vi "labHolo.vi"() -> ()   [LabVIEW 2023] (continued)
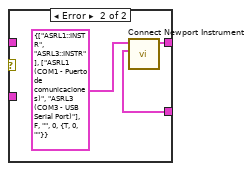
[diagram p2: hidden frame]
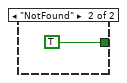
[diagram p4: hidden frame]
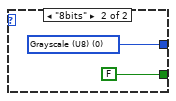
[diagram p5: hidden frame]
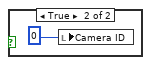
[diagram p6: hidden frame]
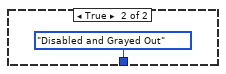
[diagram p7: hidden frame]
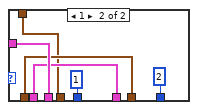
[diagram p8: hidden frame]
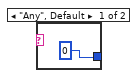
[diagram p13: hidden frame]
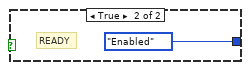
[diagram p14: hidden frame]
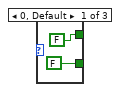
[diagram p15: hidden frame]
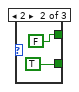
[diagram p16: hidden frame]
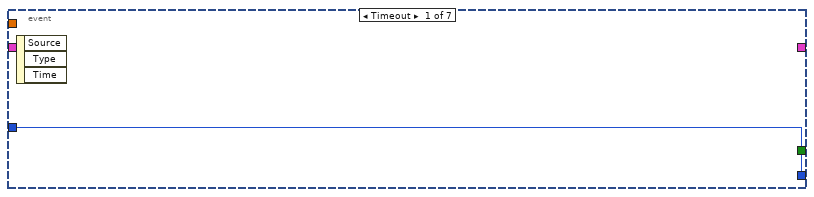
[diagram p17: hidden frame]
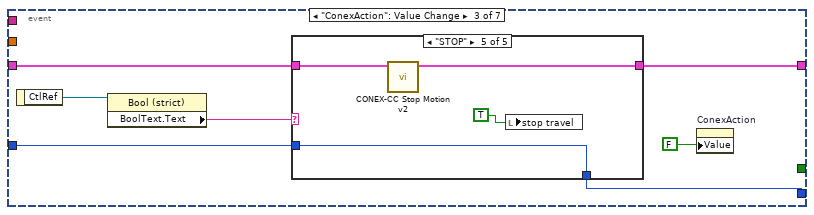
[diagram p18: hidden frame]
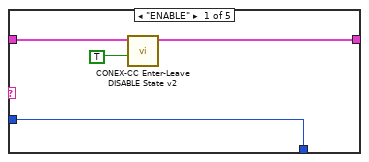
[diagram p19: hidden frame]
                n313 = Unbundle By Name(w777) -> ("1_Ygros"=w782:dbl, "1_Yfine"=w783:dbl)
                n314 = Multiply(x=w781, y=w782) -> (x*y=w780:dbl)
                n315 = Multiply(x=w783, y=w781) -> (x*y=w778:dbl)
                n316 = property on="Ygros" class="Slide (strict)"("Val(Sgnl)"=w780) -> (error out=w779:errorcluster)  [unwired: 2 in, 1 out]
                n317 = Bundle By Name(cluster=w777, "1_Ygros"=w780, "1_Yfine"=w778, "1_Yreverse"=w775) -> (w776:T4)
                n318 = property on="Yfine" class="Slide (strict)"(error in=w779, "Val(Sgnl)"=w778) -> ()  [unwired: 1 in, 2 out]
              }
            }
            n319 = case shown="1" w724 {
              tunnel: w729 -> [w733 w735]
              tunnel: w731 -> [w732 w734]
              frame 0, Default {
                n320 = local write "1_posCluster"(w733) -> ()
                n321 = local write "1_mainPos"(w732) -> ()
              }
              frame 1 {
                n322 = local write "2_posCluster"(w735) -> ()
                n323 = local write "2_mainPos"(w734) -> ()
              }
            }
          }
          event "setXi", "setXf", "setYi", "setYf": Value Change {
            w788 = FALSE ("setYf")
            n324 = event-data() -> ("CtlRef"=w787:refnum<vi>)  [unwired: 1 in, 2 out]
            n325 = case shown="0, Default" w786 {
              tunnel: [w804 w805] -> w790
              frame 0, Default {
                n326 = local read "1_mainPos"() -> (w804:T3)
              }
              frame 1 {
                n327 = local read "2_mainPos"() -> (w805:T3)
              }
            }
            n328 = property class="Bool (strict)"(reference=w787) -> ("Label.Text"=w789:string)  [unwired: 1 in, 2 out]
            n329 = local read "Ypos"() -> (w792:i32)
            n330 = local read "Xpos"() -> (w791:i32)
            n331 = case shown="\"setYf\"" w789 {
              tunnel: w790 -> [w808 w811 w813 w816 w819]
              tunnel: [w808 w810 w812 w815 w818] -> w793
              tunnel: w791 -> [_ w809 w814 _ _]
              tunnel: w792 -> [_ _ _ w817 w820]
              frame "Any", Default {
              }
              frame "setXi" {
                n332 = Bundle By Name(cluster=w811, "1_Xi"=w809) -> (w810:T3)
              }
              frame "setXf" {
                n333 = Bundle By Name(cluster=w813, "1_Xf"=w814) -> (w812:T3)
              }
              frame "setYi" {
                n334 = Bundle By Name(cluster=w816, "1_Yi"=w817) -> (w815:T3)
              }
              frame "setYf" {
                n335 = Bundle By Name(cluster=w819, "1_Yf"=w820) -> (w818:T3)
              }
            }
            n336 = Unbundle By Name(w793) -> ("1_Xi"=w795:dbl, "1_Xf"=w796:dbl, "1_Yi"=w797:dbl, "1_Yf"=w798:dbl)
            n337 = local write "setYf"(w788) -> ()
            n338 = local write "setYi"(w788) -> ()
            n339 = local write "setXf"(w788) -> ()
            n340 = local write "setXi"(w788) -> ()
            n341 = call "pos2centerRadi.vi"("pos fin"=w796, "pos init"=w795) -> ("semi diff (r)"=w802:dbl, "semi sum (C)"=w803:dbl)  [unwired: 8 in]
            n342 = call "pos2centerRadi.vi"("pos fin"=w798, "pos init"=w797) -> ("semi diff (r)"=w800:dbl, "semi sum (C)"=w801:dbl)  [unwired: 8 in]
            n343 = Divide(x=w802, y=w800) -> (x/y=w799:dbl)
            n344 = Bundle By Name(cluster=w793, "1_Xcenter"=w803, "1_Diam. X"=w802, "1_Ycenter"=w801, "1_Diam. Y"=w800, "1_Form fa."=w799) -> (w794:T3)
            n345 = local write "Form fa."(w799) -> ()
            n346 = local write "Diam. Y"(w800) -> ()
            n347 = local write "Ycenter"(w801) -> ()
            n348 = local write "Diam. X"(w802) -> ()
            n349 = local write "Xcenter"(w803) -> ()
            n350 = case shown="1" w786 {
              tunnel: w794 -> [w806 w807]
              frame 0, Default {
                n351 = local write "1_mainPos"(w806) -> ()
              }
              frame 1 {
                n352 = local write "2_mainPos"(w807) -> ()
              }
            }
          }
          event "SLM_number": Value Change {
            n353 = event-data() -> ("NewVal"=w825:u16)  [unwired: 1 in]
            n354 = case shown="1" w825 {
              tunnel: [w860 w863] -> w855
              tunnel: [w859 w862] -> w839
              tunnel: [w858 w861] -> w849
              frame 0, Default {
                n355 = local read "1_posCluster"() -> (w859:T4)
                n356 = local read "SLM1 cluster"() -> (w860:T2)
                n357 = local read "1_mainPos"() -> (w858:T3)
              }
              frame 1 {
                n358 = local read "SLM2 cluster"() -> (w863:T2)
                n359 = local read "2_posCluster"() -> (w862:T4)
                n360 = local read "2_mainPos"() -> (w861:T3)
              }
            }
            n361 = Unbundle By Name(w855) -> ("1_Radio"=w823:T7, "1_Trans"=w829:dbl, "1_Phase"=w830:dbl, "1_HoloCode"=w831:string, "1_Semi"=w832:bool, "1_Active"=w857:u16, "1_ModType"=w833:string, "1_Flip"=w834:string, "1_HoloNum"=w835:dbl, "1_key1"=w836:string, "1_value1"=w837:i64, "1_key2"=w838:string)
            n362 = Unbundle By Name(w849) -> ("1_Xcenter"=w850:dbl, "1_Ycenter"=w851:dbl, "1_Diam. X"=w852:dbl, "1_Diam. Y"=w853:dbl, "1_Form fa."=w854:dbl)
            n363 = Unbundle By Name(w839) -> ("1_Xoffset"=w840:dbl, "1_Yoffset"=w841:dbl, "1_Xgros"=w842:dbl, "1_Ygros"=w843:dbl, "1_Xfine"=w844:dbl, "1_Yfine"=w845:dbl, "1_Xreverse"=w846:u16, "1_Yreverse"=w847:u16, "1_XYswap"=w848:u16)
            n364 = local write "Radio"(w823) -> ()
            n365 = local write "Trans"(w829) -> ()
            n366 = local write "Phase"(w830) -> ()
            n367 = local write "HoloCode"(w831) -> ()
            n368 = local write "Semi"(w832) -> ()
            n369 = local write "Active"(w857) -> ()
            n370 = local write "ModType"(w833) -> ()
            n371 = local write "Flip"(w834) -> ()
            n372 = local write "HoloNum"(w835) -> ()
            n373 = local write "Xreverse"(w846) -> ()
            n374 = local write "Yreverse"(w847) -> ()
            n375 = local write "XYswap"(w848) -> ()
            n376 = local write "Xcenter"(w850) -> ()
            n377 = local write "Ycenter"(w851) -> ()
            n378 = local write "Diam. X"(w852) -> ()
            n379 = local write "Diam. Y"(w853) -> ()
            n380 = local write "Form fa."(w854) -> ()
            n381 = local write "Xoffset"(w840) -> ()
            n382 = local write "Ygros"(w843) -> ()
            n383 = local write "Xfine"(w844) -> ()
            n384 = local write "value1"(w837) -> ()
            n385 = local write "Yoffset"(w841) -> ()
            n386 = local write "Xgros"(w842) -> ()
            n387 = local write "Yfine"(w845) -> ()
            n388 = local write "key1"(w836) -> ()
            n389 = local write "key2"(w838) -> ()
            n390 = Increment(x=w825) -> (x+1=w856:u16)
            n391 = call "holoPathEditor.vi"("Display"=w856, "prev. Path"=w826, "input cluster"=w855) -> ("appended path"=w827:path)  [unwired: 5 in, 3 out]
            n392 = Unbundle(w822) -> ("New Image"=w821:T6)  [unwired: 2 out]
            n393 = call "IMAQ ReadFile"("File Path"=w827, "Image"=w821) -> ("Image Out"=w828:T6)  [unwired: 5 in, 4 out]
            n394 = property on="Active" class="Ring (strict)"("Val(Sgnl)"=w857) -> ()  [unwired: 2 in, 2 out]
          }
          event "Parada Total": Value Change {
            n395 = event-data() -> ("NewVal"=w868:bool)  [unwired: 1 in, 5 out]
            n396 = Close Python Session(session in=w864) -> ()  [unwired: 1 in, 1 out]
          }
        }
        n397 = local write "CGH path"(w559) -> ()
        n398 = local write "monitor2"(w560) -> ()
        n399 = local write "monitor1"(w560) -> ()
        "error get holo" <- w561
      }
      n400 = while {
        shift-right: [w442] -> _
        shift-left: w318 -> [w443]
        tunnel: w311 -> [w438]
        stop <- w432 stop-if-true
        # "Buttons loop"
        n401 = local read "Last mov."() -> (w439:u16)
        n402 = local read "lambda"() -> (w440:dbl)
        n403 = local read "Units"() -> (w441:string)
        n404 = event shown="[1] \"Parada Total\": Value Change" {
          selector: _ -> [_ _ _ _ _ _ _]
          dyn-events: _ -> [_ _ _ _ _ _ _]
          timeout: _ -> [_ _ _ _ _ _ _]
          tunnel: [_ w453 _ _ _ _ _] -> w432
          tunnel: w443 -> [_ w454 w472 w506 w526 w533 w544]
          tunnel: [_ w452 w471 w505 w525 w533 w544] -> w442
          tunnel: w441 -> [_ _ _ w499 w524 _ _]
          tunnel: w440 -> [_ _ _ w498 w523 _ w537]
          tunnel: [w450 w451 w467 w496 w515 w532 w536] -> w437
          tunnel: w439 -> [w450 w451 w466 _ _ w532 w536]
          tunnel: w438 -> [_ _ _ w497 _ _ _]
          event Timeout {
            n405 = event-data() -> ()  [unwired: 1 in, 3 out]
          }
          event "Parada Total": Value Change {
            n406 = event-data() -> ()  [unwired: 1 in, 1 out]
            n407 = flat-sequence {
              tunnel: [w459] -> w457
              tunnel: w454 -> [w458]
              tunnel: w457 -> [w461]
              tunnel: [w461] -> w456
              tunnel: w456 -> [w463]
              tunnel: [w463] -> w455
              tunnel: [w465] -> w452
              tunnel: w455 -> [w465]
              tunnel: [TRUE] -> w453
              frame #0 {
                n408 = call "CONEX-CC Stop Motion v2.vi"("Connection Cluster in"=w458) -> ("Connection Cluster out"=w459:T16)  [unwired: 10 in]
              }
              frame #1 {
                n409 = local write "Travel"(FALSE) -> ()
              }
              frame #2 {
                n410 = Wait (ms)(milliseconds to wait=u32 200 ("attente (ms)")) -> ()  [unwired: 1 out]
              }
              frame #3 {
              }
            }
          }
          event "ConexAction": Value Change {
            n411 = event-data() -> ("CtlRef"=w469:refnum<vi>)  [unwired: 1 in]
            n412 = property on="Property Node" class="Bool (strict)"(reference=w469) -> ("BoolText.Text"=w468:string)  [unwired: 1 in, 2 out]
            n413 = case shown="\"STOP\"" w468 {
              tunnel: w472 -> [w475 w478 w481 w489 w492]
              tunnel: [w474 w478 w480 w488 w493] -> w471
              tunnel: [w473 w477 w479 w486 w491] -> w467
              tunnel: w466 -> [w473 w477 _ w486 w491]
              frame "ENABLE" {
                n414 = call "CONEX-CC Enter-Leave DISABLE State v2.vi"("Ready? (false=DISABLE true=READY)"=TRUE ("Flag (false=DISABLE true=READY)"), "Connection Cluster in"=w475) -> ("Connection Cluster out"=w474:T16)  [unwired: 7 in]
              }
              frame Default {
              }
              frame "HOME" {
                n415 = flat-sequence {
                  tunnel: w481 -> [w485]
                  tunnel: [w484] -> w480
                  tunnel: [w483] -> w479
                  frame #0 {
                    n416 = One Button Dialog(message="The Stage will go to the 0 position. Check that the travel is clean!") -> ()  [unwired: 1 in, 1 out]
                  }
                  frame #1 {
                    w483 = u16 0 items=["opening", "homing", "toLeft", "toRight", "closing"] ("Last movement")
                    n417 = call "CONEX-CC Home search v2.vi"("Connection Cluster in"=w485) -> ("Connection Cluster out"=w484:T16)  [unwired: 5 in, 3 out]
                  }
                }
              }
              frame "DISABLE" {
                n418 = call "CONEX-CC Enter-Leave DISABLE State v2.vi"("Ready? (false=DISABLE true=READY)"=FALSE ("Flag (false=DISABLE true=READY)"), "Connection Cluster in"=w489) -> ("Connection Cluster out"=w488:T16)  [unwired: 7 in]
              }
              frame "STOP" {
                n419 = call "CONEX-CC Stop Motion v2.vi"("Connection Cluster in"=w492) -> ("Connection Cluster out"=w493:T16)  [unwired: 10 in]
                n420 = local write "stop travel"(TRUE ("stop travel")) -> ()
              }
            }
            n421 = property on="ConexAction" class="Bool (strict)"("Value"=FALSE) -> ()  [unwired: 2 in, 2 out]
          }
          event "step forward", "step backward": Value Change {
            n422 = event-data() -> ("CtlRef"=w508:refnum<vi>)  [unwired: 1 in]
            n423 = property on="Property Node" class="Bool (strict)"(reference=w508) -> (reference out=w501:refnum<vi>, error out=w503:errorcluster, "Label.Text"=w504:string)  [unwired: 1 in]
            n424 = local read "Step:"() -> (w500:dbl)
            n425 = call "step_movement.vi"("lambda (nm)"=w498, "Units"=w499, "error in (no error)"=w503, "step (units)"=w500, "Step type (fordward)"=w504, "Connection Cluster in"=w506) -> ("error out"=w502:errorcluster, "Last mov."=w496:u16, "Connection Cluster out"=w505:T16)  [unwired: 3 in]
            n426 = property on="Property Node" class="Bool (strict)"(reference=w501, error in=w502, "Value"=FALSE) -> (error out=w495:errorcluster)  [unwired: 1 out]
            n427 = local read "Travel"() -> (w494:bool)
            n428 = case shown="True" w494 {
              tunnel: w497 -> [_ w511]
              tunnel: w495 -> [_ w510]
              frame False {
              }
              frame True {
                n429 = Send Notification(notification="", notifier=w511, error in (no error)=w510) -> ()  [unwired: 2 out]
              }
            }
          }
          event "Go1", "Go2", "Go0": Value Change {
            n430 = event-data() -> ("CtlRef"=w522:refnum<vi>)  [unwired: 1 in]
            n431 = property on="Property Node" class="Bool (strict)"(reference=w522) -> (reference out=w521:refnum<vi>, "Label.Text"=w519:string)  [unwired: 1 in, 1 out]
            n432 = case shown="\"Go0\", Default" w519 {
              tunnel: [w529 w530 0.0 ("(2) Go to:")] -> w513
              frame "Go1" {
                n433 = local read "(1) Go to:"() -> (w529:dbl)
              }
              frame "Go2" {
                n434 = local read "(2) Go to:"() -> (w530:dbl)
              }
              frame "Go0", Default {
              }
            }
            n435 = local read "Zero pos."() -> (w514:dbl)
            n436 = Add(x=w514, y=w513) -> (x+y=w512:dbl)
            n437 = local read "Relative pos."() -> (w517:dbl)
            n438 = call "units2mm.vi"("lambda (nm)"=w523, "target units"=w524, "position in units"=w512) -> ("raw postion (mm)"=w518:dbl)  [unwired: 8 in]
            n439 = property on="Property Node" class="Bool (strict)"(reference=w521, "Value"=FALSE) -> ()  [unwired: 1 in, 2 out]
            n440 = Greater?(x=w518, y=w517) -> (0:w516:bool)
            n441 = case shown="False" w516 {
              tunnel: [w527 w528] -> w515
              frame False {
                w527 = u16 2 items=["opening", "homing", "toLeft", "toRight", "closing"] ("Last movement")
              }
              frame True {
                w528 = u16 3 items=["opening", "homing", "toLeft", "toRight", "closing"] ("Last movement")
              }
            }
            n442 = call "CONEX-CC Absolute Move v2.vi"("Target position"=w518, "Connection Cluster in"=w526) -> ("Connection Cluster out"=w525:T16)  [unwired: 5 in, 2 out]
          }
          event "Tare": Value Change {
            n443 = event-data() -> ()  [unwired: 1 in, 2 out]
            n444 = local read "Raw position"() -> (w535:dbl)
            n445 = local write "Tare"(FALSE ("Tare")) -> ()
            n446 = local write "Zero pos."(w535) -> ()
          }
          event "Units": Value Change {
            n447 = event-data() -> ("OldVal"=w543:string, "NewVal"=w545:string)  [unwired: 1 in]
            n448 = property on="(1) Go to:" class="DigNum (strict)"("Caption.Text"=w545) -> ()  [unwired: 2 in, 2 out]
            n449 = property on="(2) Go to:" class="DigNum (strict)"("Caption.Text"=w545) -> ()  [unwired: 2 in, 2 out]
            n450 = property on="Zero pos." class="DigNum (strict)"("Caption.Text"=w545) -> ()  [unwired: 2 in, 2 out]
            n451 = property on="Raw position" class="DigNum (strict)"("Caption.Text"=w545) -> ()  [unwired: 2 in, 2 out]
            n452 = property on="Relative pos." class="DigNum (strict)"("Caption.Text"=w545) -> ()  [unwired: 2 in, 2 out]
            n453 = property on="Step:" class="DigNum (strict)"("Caption.Text"=w545) -> ()  [unwired: 2 in, 2 out]
            n454 = case shown="\"lam\"" w543 {
              tunnel: [1000000.0 1000.0 1.0 w549] -> w539
              tunnel: w537 -> [_ _ _ w549]
              frame "mm", Default {
              }
              frame "um" {
              }
              frame "nm" {
              }
              frame "lam" {
              }
            }
            n455 = case shown="\"lam\"" w545 {
              tunnel: [1000000.0 1000.0 1.0 w553] -> w538
              tunnel: w537 -> [_ _ _ w553]
              frame "mm", Default {
              }
              frame "um" {
              }
              frame "nm" {
              }
              frame "lam" {
              }
            }
            n456 = local read "Zero pos."() -> (w542:dbl)
            n457 = Divide(x=w539, y=w538) -> (x/y=w540:dbl)
            n458 = Multiply(x=w542, y=w540) -> (x*y=w541:dbl)
            n459 = local write "Zero pos."(w541) -> ()
          }
        }
        n460 = case shown="3" w437 {
          tunnel: [FALSE ("Boolean Text.Font:Bold") FALSE ("Boolean Text.Font:Bold") TRUE ("Boolean Text.Font:Bold")] -> w435
          tunnel: [FALSE ("Boolean Text.Font:Bold") TRUE ("Boolean Text.Font:Bold") FALSE ("Boolean Text.Font:Bold")] -> w436
          frame 0, Default {
          }
          frame 2 {
          }
          frame 3 {
          }
        }
        n461 = Not(x=w432) -> (.not. x?=w431:bool)
        n462 = local write "Last mov."(w437) -> ()
        n463 = And(x=w435, y=w431) -> (x .and. y?=w434:bool)
        n464 = And(x=w436, y=w431) -> (x .and. y?=w433:bool)
        n465 = property on="step backward" class="Bool (strict)"("BoolText.FontUnder"=w433) -> ()  [unwired: 2 in, 2 out]
        n466 = property on="step forward" class="Bool (strict)"("BoolText.FontUnder"=w434) -> ()  [unwired: 2 in, 2 out]
      }
      n467 = while {
        shift-right: [w884] -> _
        shift-left: _ -> [w883]
        tunnel: w330 -> [w881]
        tunnel: w305 -> [w880]
        tunnel: w329 -> [w878]
        tunnel: w328 -> [w877]
        shift-right: [w873] -> _
        shift-left: w327 -> [w875]
        shift-right: [w872] -> _
        shift-left: w326 -> [w874]
        tunnel: w325 -> [w871]
        tunnel: w309 -> [w870]
        tunnel: w310 -> [w869]
        stop <- w885 stop-if-true
        # "Cam control"
        # "pyError"
        # "Reff"
        # "ROI"
        # "CCD"
        # "pySession"
        n468 = local read "Camera ID"() -> (w876:u16)
        n469 = event shown="[0] Timeout" {
          selector: _ -> [_ _ _ _ _ _ _]
          dyn-events: _ -> [_ _ _ _ _ _ _]
          timeout: 10 -> [_ _ _ _ _ _ _]
          tunnel: [_ _ _ _ _ _ w1053] -> w885
          tunnel: [w912 _ _ _ _ _ _] -> w884
          tunnel: w883 -> [w920 _ _ _ _ _ _]
          tunnel: w881 -> [w918 _ _ w963 _ _ _]
          tunnel: w880 -> [w917 _ _ w962 w1005 _ w1052]
          tunnel: [w916 _ _ w961 w1003 _ w1050] -> w879
          tunnel: w878 -> [w901 _ _ _ _ _ _]
          tunnel: w877 -> [w900 _ _ _ _ _ _]
          tunnel: w876 -> [w902 _ _ _ w994 _ _]
          tunnel: w875 -> [w897 _ _ _ _ _ _]
          tunnel: w874 -> [w896 _ _ _ _ _ _]
          tunnel: [w895 _ _ _ _ _ _] -> w873
          tunnel: [w894 _ _ _ _ _ _] -> w872
          tunnel: w871 -> [w892 _ _ w959 w993 _ w1051]
          tunnel: w870 -> [_ _ _ w956 _ _ _]
          tunnel: w869 -> [_ _ _ w954 _ _ _]
          event Timeout {
            n470 = event-data() -> ()  [unwired: 1 in, 3 out]
            n471 = call "capture.vi"("error in (no error)"=w892, "Cam ID"=w902, "Image in"=w918, "session in"=w917) -> ("error out"=w916:errorcluster, "Image out"=w899:T6)  [unwired: 3 in, 1 out]
            n472 = local read "bit depth"() -> (w906:enum16{"16bits", "14bits", "12bits", "8bits"})
            n473 = property on="CCD Image" class="ImageControl"() -> ("ROI"=w886:T8)  [unwired: 2 in, 2 out]
            "ROI" <- w886
            n474 = call "histogram.vi"("Image ROI"=w900, "useROI"="Whole/ROI", "ROI Descriptor"=w886, "bit depth"=w906, "Image"=w899) -> ("Statistics"=w909:T20, "Histograph"=→"Histograph":T9, "bins"=w898:i32)  [unwired: 2 in, 2 out]
            n475 = Unbundle By Name(w909) -> ("mean (ROI)"=w889:dbl, "max (ROI)"=w888:i16, "max_counts"=w908:dbl, "image_size"=→"ROI size":i32, "# Sat. Pixels"=w887:sgl)
            "mean bar" <- w889
            "mean" <- w889
            "max" <- w888
            "# Sat. Pixels" <- w887
            n476 = control-ref of="Histograph"() -> (w907:refnum<vi>)
            n477 = control-ref of="Reff ROI"() -> (w910:refnum<vi>)
            n478 = call "setHistogram.vi"("Auto. In"="Auto. hist", "max counts"=w908, "bins"=w898, "WaveformGraph in"=w907) -> ()  [unwired: 7 in, 1 out]
            n479 = call "drawRoi.vi"("bit depth"=w906, "ROI"=w910, "Reff image"=w901, "Whole image"=w899) -> ("size"=→"size":i32, "mean"=w905:dbl, "Image Out"=w891:T6, "Percentile alert"=w893:bool)  [unwired: 3 in, 1 out]
            "CCD Image" <- w891
            n480 = Tick Count (ms)() -> (millisecond timer value=w912:u32)
            n481 = Subtract(x=w912, y=w920) -> (x-y=w923:u32)
            n482 = case shown="True" "EnlargeCCD" {
              tunnel: w891 -> [_ w928]
              tunnel: w889 -> [_ w927]
              tunnel: w888 -> [_ w926]
              tunnel: w887 -> [_ w925]
              tunnel: w886 -> [_ w924]
              frame False {
              }
              frame True {
                n483 = call "showCCD_dedicatedWindow.vi"("ROI Descriptor"=w924, "# Sat. Pix."=w925, "Max"=w926, "Mean"=w927, "Refnum in"=w928) -> ()  [unwired: 7 in]
              }
            }
            n484 = Reciprocal(x=w923) -> (1/x=w922:dbl)
            n485 = call "meanAndVar.vi"("new mean value"=w905, "MEAN array in"=w897, "VAR array in"=w896) -> ("arrays stack"=→"Chart TimeSeries":dbl[][], "MEAN array out"=w895:dbl[], "VAR array out"=w894:dbl[])  [unwired: 2 in]
            n486 = Multiply(x=u32 1000 ("y"), y=w922) -> (x*y=→"Real FPS":dbl)
            n487 = property on="Reff alert" class="Bool (strict)"("Blinking"=w893) -> ()  [unwired: 2 in, 2 out]
          }
          event "Zoom2Fit", "EnlargeCCD": Value Change {
            n488 = event-data() -> ("CtlRef"=w932:refnum<vi>, "NewVal"=w930:bool)  [unwired: 1 in, 4 out]
            n489 = property class="Bool (strict)"(reference=w932) -> ("Label.Text"=w931:string)  [unwired: 1 in, 2 out]
            n490 = case shown="\"EnlargeCCD\", Default" w931 {
              tunnel: w930 -> [w934 w945]
              tunnel: 9 ("Window Number (0...15)") -> [w933 w944]
              frame "EnlargeCCD", Default {
                n491 = case shown="True" w934 {
                  tunnel: w933 -> [w937 w942]
                  frame False {
                    n492 = call "IMAQ WindClose"("Window Number (0...15)"=w937) -> ("error out"=w936:errorcluster)  [unwired: 5 in]
                    n493 = property on="Zoom2Fit" class="Bool (strict)"("DisabledEnum"=T10."Disabled and Grayed Out" ("Disabled")) -> ()  [unwired: 2 in, 2 out]
                    n494 = call "IMAQ WindToolsClose"("error in (no error)"=w936) -> ()  [unwired: 5 in, 1 out]
                  }
                  frame True {
                    w941 = 1 items=["Hide", "Show", "No change"] ("Scrollbars (No change)")
                    n495 = call "IMAQ WindSetup"("Scrollbars (No change)"=w941, "Window is floating? (No)"=TRUE, "Window Number (0...15)"=w942, "Window can close? (Yes)"=FALSE) -> ()  [unwired: 7 in, 1 out]
                    n496 = property on="Zoom2Fit" class="Bool (strict)"("Visible"=TRUE, "DisabledEnum"=T10."Enabled" ("Disabled")) -> ()  [unwired: 2 in, 2 out]
                  }
                }
              }
              frame "Zoom2Fit" {
                n497 = call "IMAQ WindZoom 2"("Window Number (0...15)"=w944, "Zoom to Fit? (False)"=w945) -> ()  [unwired: 6 in, 4 out]
              }
            }
            n498 = call "IMAQ WindLastEvent"() -> ()  [unwired: 6 in, 6 out]
          }
          event "take reff", "Reset reff.": Value Change {
            w949 = dbl[] [] ("RefTimeSeries")
            w948 = FALSE ("take reff")
            n499 = event-data() -> ("CtlRef"=w947:refnum<vi>)  [unwired: 1 in, 5 out]
            n500 = property class="Bool (strict)"(reference=w947) -> ("Label.Text"=w946:string)  [unwired: 1 in, 2 out]
            n501 = case shown="\"take reff\"" w946 {
              frame "Any", Default {
              }
              frame "take reff" {
                n502 = property on="CCD Image" class="ImageControl"() -> ("ROI"=→"Reff ROI":T8)  [unwired: 2 in, 2 out]
              }
            }
            n503 = local write "Reset reff."(w948) -> ()
            n504 = local write "take reff"(w948) -> ()
            n505 = local write "Mean array"(w949) -> ()
            n506 = local write "Var array"(w949) -> ()
          }
          event "suffix", "Polarizer", "Analyzer", "beam_name", "Save": Value Change {
            n507 = event-data() -> ("CtlRef"=w965:refnum<vi>)  [unwired: 1 in, 5 out]
            n508 = local read "Travel"() -> (w952:bool)
            n509 = property class="Ctl"(reference=w965, error in=w959) -> (reference out=w960:refnum<vi>, error out=w958:errorcluster, "Label.Text"=w964:string)
            n510 = local read "beam_name"() -> (w969:string)
            n511 = case shown="True" w952 {
              tunnel: w954 -> [_ w972]
              tunnel: [w970 w971] -> w953
              frame False {
                n512 = local read "suffix"() -> (w970:string)
              }
              frame True {
                n513 = Wait on Notification with Notifier History(0:w972) -> (9:w971:string)  [unwired: 3 in, 3 out]
                n514 = local write "suffix"(w971) -> ()
              }
            }
            n515 = local read "Polarizer"() -> (w968:string)
            n516 = local read "Analyzer"() -> (w967:string)
            n517 = local read "key2"() -> (w966:string)
            n518 = local read "Active"() -> (w951:u16)
            n519 = call "getSavePath.vi"("beam_name"=w969, "Polarizer"=w968, "Analyzer"=w967, "prefix"=w966, "suffix"=w953, "active"=w951) -> ("appended filename"=w957:string)  [unwired: 9 in]
            n520 = case shown="\"Save\"" w964 {
              tunnel: w957 -> [w973 w990]
              tunnel: w963 -> [_ w992]
              tunnel: w962 -> [_ w991]
              tunnel: [errorcluster {"status"=FALSE, "code"=0, "source"=""} ("error out") w980] -> w961
              tunnel: w960 -> [_ w984]
              tunnel: w958 -> [_ w985]
              tunnel: [w973 w986] -> w955
              tunnel: w952 -> [_ w976]
              frame "Any", Default {
              }
              frame "Save" {
                n521 = property on="Property Node" class="Ctl"(reference=w984, error in=w985, "DisabledEnum"=T10."Disabled and Grayed Out" ("Disabled")) -> (reference out=w983:refnum<vi>, error out=w982:errorcluster)
                n522 = Not(x=w976) -> (.not. x?=w975:bool)
                n523 = local read "Reff ROI"() -> (w988:T8)
                n524 = local read "bit depth"() -> (w987:enum16{"16bits", "14bits", "12bits", "8bits"})
                n525 = property on="CCD Image" class="ImageControl"() -> ("ROI"=w989:T8)  [unwired: 2 in, 2 out]
                n526 = call "saveImage.vi"("UserDialog"=w975, "error in"=w982, "bit depth"=w987, "session in"=w991, "Reff ROI"=w988, "main ROI"=w989, "appended filename"=w990, "Image in"=w992) -> ("error out"=w981:errorcluster, "png filename"=w986:string)  [unwired: 2 out]
                n527 = property on="Property Node" class="Ctl"(reference=w983, error in=w981, "DisabledEnum"=T10."Enabled" ("Disabled"), "Value"=FALSE ("Save")) -> (error out=w980:errorcluster)  [unwired: 1 out]
              }
            }
            n528 = local write "default filename"(w957) -> ()
            n529 = Send Notification(notification=w955, notifier=w956) -> ()  [unwired: 1 in, 2 out]
          }
          event "FPS", "Exposure (ms)", "Gain": Value Change {
            n530 = event-data() -> ("CtlRef"=w1001:refnum<vi>, "NewVal"=w1004:dbl)  [unwired: 1 in, 4 out]
            n531 = property class="DigNum (strict)"(reference=w1001) -> ("Label.Text"=w1002:string)  [unwired: 1 in, 2 out]
            n532 = case shown="\"FPS\"" w1002 {
              tunnel: w1005 -> [w1012 w1019 w1028]
              tunnel: w1004 -> [w1011 w1018 w1020]
              tunnel: [w1010 w1017 w1026] -> w1003
              tunnel: w994 -> [w1007 w1016 w1021]
              tunnel: [w1008 w1015 w1025] -> w996
              tunnel: [w1009 w1014 w1024] -> w995
              tunnel: w993 -> [w1006 w1013 w1027]
              frame "Exposure (ms)", Default {
                n533 = call "set_exposure.vi"("error in (no error)"=w1006, "cam ID"=w1007, "exposure"=w1011, "Session in"=w1012) -> ("error out"=w1010:errorcluster, "true FPS"=w1008:dbl, "true exposure"=w1009:dbl)  [unwired: 3 in, 1 out]
              }
              frame "FPS" {
                n534 = call "set_fps.vi"("error in (no error)"=w1013, "cam ID"=w1016, "FPS"=w1018, "Session in"=w1019) -> ("error out"=w1017:errorcluster, "true Exposure"=w1014:dbl, "true FPS"=w1015:dbl)  [unwired: 3 in, 1 out]
              }
              frame "Gain" {
                n535 = local read "gains"() -> (w1023:dbl[])
                n536 = call "set_gain.vi"("error in (no error)"=w1027, "cam ID"=w1021, "Gain"=w1020, "Session in"=w1028) -> ("error out"=w1026:errorcluster, "true Exposure"=w1024:dbl, "true FPS"=w1025:dbl)  [unwired: 3 in, 1 out]
                n537 = Replace Array Subset(array=w1023, new element=w1020, index=w1021) -> (w1022:dbl[])
                n538 = local write "gains"(w1022) -> ()
              }
            }
            n539 = local write "Exposure (ms)"(w995) -> ()
            n540 = local write "FPS"(w996) -> ()
            n541 = local read "exposures"() -> (w999:dbl[])
            n542 = local read "FPSs"() -> (w1000:dbl[])
            n543 = Replace Array Subset(array=w999, new element=w995, index=w994) -> (w997:dbl[])
            n544 = Replace Array Subset(array=w1000, new element=w996, index=w994) -> (w998:dbl[])
            n545 = local write "exposures"(w997) -> ()
            n546 = local write "FPSs"(w998) -> ()
          }
          event "Camera ID": Value Change {
            n547 = event-data() -> ("OldVal"=w1030:u16, "NewVal"=w1029:u16)  [unwired: 1 in, 4 out]
            n548 = flat-sequence {
              tunnel: w1030 -> [w1031]
              tunnel: w1029 -> [w1043]
              frame #0 {
                n549 = local read "Exposure (ms)"() -> (w1040:dbl)
                n550 = local read "gains"() -> (w1034:dbl[])
                n551 = local read "FPSs"() -> (w1035:dbl[])
                n552 = local read "Gain"() -> (w1032:dbl)
                n553 = local read "exposures"() -> (w1039:dbl[])
                n554 = local read "FPS"() -> (w1037:dbl)
                n555 = Replace Array Subset(array=w1034, new element=w1032, index=w1031) -> (w1033:dbl[])
                n556 = Replace Array Subset(array=w1039, new element=w1040, index=w1031) -> (w1038:dbl[])
                n557 = Replace Array Subset(array=w1035, new element=w1037, index=w1031) -> (w1036:dbl[])
                n558 = local write "exposures"(w1038) -> ()
                n559 = local write "FPSs"(w1036) -> ()
                n560 = local write "gains"(w1033) -> ()
              }
              frame #1 {
                n561 = local read "exposures"() -> (w1049:dbl[])
                n562 = local read "FPSs"() -> (w1048:dbl[])
                n563 = local read "gains"() -> (w1042:dbl[])
                n564 = Index Array(array=w1048, index=w1043) -> (element=w1047:dbl)
                n565 = Index Array(array=w1049, index=w1043) -> (element=w1046:dbl)
                n566 = Index Array(array=w1042, index=w1043) -> (element=w1041:dbl)
                n567 = property on="FPS" class="DigNum (strict)"("Val(Sgnl)"=w1047) -> (error out=w1045:errorcluster)  [unwired: 2 in, 1 out]
                n568 = property on="Exposure (ms)" class="DigNum (strict)"(error in=w1045, "Val(Sgnl)"=w1046) -> (error out=w1044:errorcluster)  [unwired: 1 in, 1 out]
                n569 = property on="Gain" class="DigNum (strict)"(error in=w1044, "Val(Sgnl)"=w1041) -> ()  [unwired: 1 in, 2 out]
              }
            }
          }
          event "Parada Total": Value Change {
            n570 = event-data() -> ("NewVal"=w1053:bool)  [unwired: 1 in, 5 out]
            n571 = Close Python Session(session in=w1052, error in=w1051) -> (11:w1050:errorcluster)
          }
        }
        "py error" <- w879
      }
      n572 = timed-loop {
        timing: w321 -> [_]
        timing-out: [_] -> w320
        shift-right: [w410] -> w319
        shift-left: w318 -> [w416]
        tunnel: w306 -> [w396]
        stop <- w411 stop-if-true
        # "Working loop"
        n573 = node-c288() -> ()  [unwired: 2 out]
        n574 = call "CONEX-CC Get Current Position v2.vi"("Connection Cluster in"=w416) -> ("Current position"=w407:dbl, "Connection Cluster out"=w415:T16)  [unwired: 8 in, 1 out]
        n575 = local read "Travel"() -> (w400:bool)
        n576 = call "CONEX-CC Get Positioner Error And Controller State v2.vi"("Connection Cluster in"=w415) -> ("Controller state"=w413:string, "Positioner error"=w414:string, "Connection Cluster out"=w410:T16)  [unwired: 8 in]
        n577 = Not(x=w400) -> (.not. x?=w401:bool)
        n578 = call "Get Positioner Error And Controller State Descriptions.vi"("Controller state"=w413, "Positioner error"=w414) -> ("Color"=w419:u32, "Action name"=w404:string, "Controller state description"=→"Controller state description":string, "IsReady?"=w399:bool)  [unwired: 2 out]
        "ConexCC ready" <- w399
        n579 = And(x=w401, y=w399) -> (x .and. y?=w402:bool)
        n580 = property on="ConexAction" class="Bool (strict)"("BoolText.Text"=w404) -> ()  [unwired: 2 in, 2 out]
        n581 = property on="Controller state description" class="Str"("Text.FontColor"=w419) -> ()  [unwired: 2 in, 2 out]
        n582 = case shown="False" w402 {
          tunnel: [T10."Disabled and Grayed Out" ("Disabled") T10."Enabled" ("Disabled")] -> w405
          frame False {
            # "MOVING"
          }
          frame True {
            # "READY"
          }
        }
        n583 = String Length(string=w404) -> (length=w418:i32)
        n584 = case shown="\"DISABLE\"" w404 {
          tunnel: [0 2] -> w403
          frame "Any", Default {
          }
          frame "DISABLE" {
          }
        }
        n585 = Greater Than 0?(x=w418) -> (x > 0?=w417:bool)
        n586 = property on="ConexAction" class="Bool (strict)"("DisabledEnum"=w403, "Visible"=w417) -> ()  [unwired: 2 in, 2 out]
        n587 = property on="Go0" class="Bool (strict)"("Disabled"=w405) -> ()  [unwired: 2 in, 2 out]
        n588 = property on="Go1" class="Bool (strict)"("Disabled"=w405) -> ()  [unwired: 2 in, 2 out]
        n589 = property on="Go2" class="Bool (strict)"("Disabled"=w405) -> ()  [unwired: 2 in, 2 out]
        n590 = property on="Units" class="CmbBox"("Disabled"=w405) -> ()  [unwired: 2 in, 2 out]
        n591 = property on="Tare" class="Bool (strict)"("Disabled"=w405) -> ()  [unwired: 2 in, 2 out]
        n592 = property on="Travel" class="Bool (strict)"("Disabled"=w405) -> ()  [unwired: 2 in, 2 out]
        n593 = property on="step forward" class="Bool (strict)"("Disabled"=w405) -> ()  [unwired: 2 in, 2 out]
        n594 = property on="step backward" class="Bool (strict)"("Disabled"=w405) -> ()  [unwired: 2 in, 2 out]
        n595 = property on="SaveTravel" class="Bool (strict)"("Disabled"=w405) -> ()  [unwired: 2 in, 2 out]
        n596 = local read "Units"() -> (w409:string)
        n597 = local read "lambda"() -> (w408:dbl)
        n598 = call "mm2units.vi"("lambda (nm)"=w408, "target units"=w409, "raw position (mm)"=w407) -> ("position in units"=w406:dbl)  [unwired: 8 in]
        n599 = local read "Zero pos."() -> (w412:dbl)
        n600 = local read "Travel"() -> (w398:bool)
        n601 = local write "Raw position"(w406) -> ()
        n602 = Subtract(x=w406, y=w412) -> (x-y=w397:dbl)
        n603 = local write "Relative pos."(w397) -> ()
        n604 = case shown="True" w398 {
          tunnel: w397 -> [_ w422]
          tunnel: w396 -> [_ w421]
          frame False {
          }
          frame True {
            n605 = Send Notification(notification=w422, notifier=w421) -> ()  [unwired: 1 in, 2 out]
          }
        }
        n606 = local read "Parada Total"() -> (w411:bool)
        n607 = node-c288() -> ()  [unwired: 2 out]
      }
      n608 = node-c288(w320) -> ()  [unwired: 1 out]
    }
    frame #3 {
      w1058 = FALSE ("Visible")
      n609 = Unbundle By Name(w1060) -> ("VISA resource name"=w1062:refnum<visa-resource-name>, "error"=w1061:errorcluster)
      n610 = Release Notifier(notifier=w1056) -> ()  [unwired: 2 in, 3 out]
      n611 = Release Notifier(notifier=w1054) -> ()  [unwired: 2 in, 3 out]
      n612 = Release Notifier(notifier=w1055) -> (error out=→"error out  (Notifier)":errorcluster)  [unwired: 2 in, 2 out]
      n613 = Release Notifier(notifier=w1057) -> ()  [unwired: 2 in, 3 out]
      n614 = property on="Parada Total" class="Bool (strict)"("Value"=FALSE ("Parada Total")) -> ()  [unwired: 2 in, 2 out]
      n615 = call "IMAQ WindClose"("Close All Windows (False)"=TRUE) -> ()  [unwired: 5 in, 1 out]
      n616 = property on="stop travel" class="Bool (strict)"("Visible"=w1058, "Value"=w1058) -> ()  [unwired: 2 in, 2 out]
      n617 = call <vilib>:"Simple Error Handler.vi"("error in (no error)"=w1061) -> ()  [unwired: 1 in, 8 out]
      n618 = call "_Close Communications.vi"("Instrument Channel"=w1062) -> ()  [unwired: 14 in, 1 out]
    }
  }
